vi "15-12-13 UHR-Fleezers Control (host) - 15.2.1UCB Darwin.vi"() -> ()   [LabVIEW 2014] (continued)
            n1711 = Reciprocal(x="Flush rate (uL/m) P3") -> (1/x=w2555:dbl)
            n1712 = Number To Decimal String(number="Volume (uL) P3") -> (decimal integer string=w2560:string)  [unwired: 1 in]
            n1713 = Multiply(x="Volume (uL) P3", y=w2555) -> (x*y=w2554:dbl)
            n1714 = Concatenate Strings("tvolume  " ("string"), w2560, " u" ("string"), "\r") -> (w2558:string)
            n1715 = Multiply(x=w2554, y=60.0) -> (x*y=→"HP3 Flush Time (s)":dbl)
            n1716 = VISA Write(VISA resource name=w2569, write buffer=w2558) -> (VISA resource name out=w2557:refnum<visa-resource-name>)  [unwired: 1 in, 2 out]
            n1717 = Concatenate Strings("cvolume" ("string"), "\r") -> (w2556:string)
            n1718 = VISA Write(VISA resource name=w2557, write buffer=w2556) -> (VISA resource name out=w2567:refnum<visa-resource-name>)  [unwired: 1 in, 2 out]
            n1719 = Concatenate Strings("irun" ("string"), "\r") -> (w2565:string)
            n1720 = VISA Write(VISA resource name=w2567, write buffer=w2565) -> ()  [unwired: 1 in, 3 out]
          }
          frame #1 {
            "Flushing P3" <- TRUE ("Flushing P3")
          }
        }
        n1721 = local read "Save Event Log?"() -> (w2534:bool)
        n1722 = local read "Saving..."() -> (w2535:bool)
        n1723 = And(x=w2534, y=w2535) -> (x .and. y?=w2533:bool)
        n1724 = case shown="True" w2533 {
          tunnel: w2532 -> [_ w2539]
          tunnel: w2531 -> [_ w2538]
          frame False {
          }
          frame True {
            n1725 = Number To Decimal String(number=w2538) -> (decimal integer string=w2543:string)  [unwired: 1 in]
            n1726 = Number To Decimal String(number=w2539) -> (decimal integer string=w2545:string)  [unwired: 1 in]
            n1727 = local read "log file ref"() -> (w2540:refnum<file>)
            n1728 = local read "Time (s)"() -> (w2541:dbl)
            n1729 = Concatenate Strings("pump 3 flushing ", w2543, " uL at ", w2545, " ul/min") -> (w2547:string)
            n1730 = call "write to event log.vi"("log file ref"=w2540, "time"=w2541, "input string"=w2547) -> ()  [unwired: 8 in]
          }
        }
      }
      event "Flush Pump 1": Value Change {
        n1731 = event-data() -> ()  [unwired: 7 out]
        n1732 = flat-sequence {
          tunnel: [w2602] -> w2582
          tunnel: w2581 -> [w2597]
          tunnel: ["Volume (uL) P1"] -> w2577
          tunnel: ["Flush rate (uL/m) P1"] -> w2576
          tunnel: w2582 -> [_]
          frame #0 {
            # "set paramaters (rate, volume) for flush, clear volume"
            n1733 = local write "Inject Pump 1"(TRUE ("Inject Pump 1")) -> ()
            n1734 = Number To Decimal String(number="Flush rate (uL/m) P1") -> (decimal integer string=w2618:string)  [unwired: 1 in]
            n1735 = Concatenate Strings("irate  " ("string"), w2618, " u/m" ("string"), "\r") -> (w2620:string)
            n1736 = VISA Write(VISA resource name=w2597, write buffer=w2620) -> (VISA resource name out=w2616:refnum<visa-resource-name>)  [unwired: 1 in, 2 out]
            n1737 = Reciprocal(x="Flush rate (uL/m) P1") -> (1/x=w2601:dbl)
            n1738 = Number To Decimal String(number="Volume (uL) P1") -> (decimal integer string=w2607:string)  [unwired: 1 in]
            n1739 = Multiply(x="Volume (uL) P1", y=w2601) -> (x*y=w2600:dbl)
            n1740 = Concatenate Strings("tvolume  " ("string"), w2607, " u" ("string"), "\r") -> (w2605:string)
            n1741 = Multiply(x=w2600, y=60.0) -> (x*y=→"HP1 Flush Time (s)":dbl)
            n1742 = VISA Write(VISA resource name=w2616, write buffer=w2605) -> (VISA resource name out=w2604:refnum<visa-resource-name>)  [unwired: 1 in, 2 out]
            n1743 = Concatenate Strings("cvolume" ("string"), "\r") -> (w2603:string)
            n1744 = VISA Write(VISA resource name=w2604, write buffer=w2603) -> (VISA resource name out=w2614:refnum<visa-resource-name>)  [unwired: 1 in, 2 out]
            n1745 = Concatenate Strings("irun" ("string"), "\r") -> (w2612:string)
            n1746 = VISA Write(VISA resource name=w2614, write buffer=w2612) -> (VISA resource name out=w2602:refnum<visa-resource-name>)  [unwired: 1 in, 2 out]
          }
          frame #1 {
            "Flushing P1" <- TRUE ("Flushing P3")
          }
        }
        n1747 = local read "Saving..."() -> (w2578:bool)
        n1748 = local read "Save Event Log?"() -> (w2579:bool)
        n1749 = And(x=w2579, y=w2578) -> (x .and. y?=w2580:bool)
        n1750 = case shown="True" w2580 {
          tunnel: w2577 -> [_ w2586]
          tunnel: w2576 -> [_ w2585]
          frame False {
          }
          frame True {
            n1751 = Number To Decimal String(number=w2586) -> (decimal integer string=w2590:string)  [unwired: 1 in]
            n1752 = Number To Decimal String(number=w2585) -> (decimal integer string=w2588:string)  [unwired: 1 in]
            n1753 = local read "log file ref"() -> (w2592:refnum<file>)
            n1754 = local read "Time (s)"() -> (w2593:dbl)
            n1755 = Concatenate Strings("pump 1 flushing ", w2590, " uL at ", w2588, " ul/min") -> (w2584:string)
            n1756 = call "write to event log.vi"("log file ref"=w2592, "time"=w2593, "input string"=w2584) -> ()  [unwired: 8 in]
          }
        }
      }
      event "Clear Volume": Value Change {
        n1757 = event-data() -> ()  [unwired: 7 out]
        n1758 = Concatenate Strings("cvolume" ("string"), "\r") -> (w2624:string)
        n1759 = VISA Write(VISA resource name=w2623, write buffer=w2624) -> ()  [unwired: 1 in, 3 out]
      }
      event "Clear Volume P3": Value Change {
        n1760 = event-data() -> ()  [unwired: 7 out]
        n1761 = Concatenate Strings("cvolume" ("string"), "\r") -> (w2630:string)
        n1762 = VISA Write(VISA resource name=w2629, write buffer=w2630) -> ()  [unwired: 1 in, 3 out]
        n1763 = local write "Clear Volume P3"(FALSE ("Clear Volume P3")) -> ()
      }
      event "Clear Volume P1": Value Change {
        n1764 = event-data() -> ()  [unwired: 7 out]
        n1765 = Concatenate Strings("cvolume" ("string"), "\r") -> (w2635:string)
        n1766 = local write "Clear Volume P1"(FALSE ("Clear Volume P1")) -> ()
        n1767 = VISA Write(VISA resource name=w2634, write buffer=w2635) -> ()  [unwired: 1 in, 3 out]
      }
      event "Display On P3": Value Change {
        n1768 = event-data() -> ()  [unwired: 7 out]
        n1769 = Select(t="dim 100", s="Display On P3", f="dim 0") -> (s? t:f=w2641:string)
        n1770 = Concatenate Strings(w2641, "\r") -> (w2643:string)
        n1771 = VISA Write(VISA resource name=w2638, write buffer=w2643) -> ()  [unwired: 1 in, 3 out]
      }
      event "Display On P1": Value Change {
        n1772 = event-data() -> ()  [unwired: 7 out]
        n1773 = Select(t="dim 100", s="Display On P1", f="dim 0") -> (s? t:f=w2648:string)
        n1774 = Concatenate Strings(w2648, "\r") -> (w2650:string)
        n1775 = VISA Write(VISA resource name=w2645, write buffer=w2650) -> ()  [unwired: 1 in, 3 out]
      }
      event "Retract Pump 3": Value Change {
        n1776 = event-data() -> ()  [unwired: 7 out]
        n1777 = local write "Retract Pump 3"(FALSE ("Retract Pump 3")) -> ()
        n1778 = case shown="True" "Retract Pump 3" {
          tunnel: w2652 -> [_ w2655]
          frame False {
          }
          frame True {
            n1779 = Number To Decimal String(number="Retract Rate (uL/m)") -> (decimal integer string=w2673:string)  [unwired: 1 in]
            n1780 = Concatenate Strings("wrate  " ("string"), w2673, " u/m" ("string"), "\r") -> (w2675:string)
            n1781 = VISA Write(VISA resource name=w2655, write buffer=w2675) -> (VISA resource name out=w2666:refnum<visa-resource-name>)  [unwired: 1 in, 2 out]
            n1782 = Number To Decimal String(number="Retract Vol 3 (uL)") -> (decimal integer string=w2668:string)  [unwired: 1 in]
            n1783 = Concatenate Strings("tvolume  " ("string"), w2668, " u" ("string"), "\r") -> (w2665:string)
            n1784 = VISA Write(VISA resource name=w2666, write buffer=w2665) -> (VISA resource name out=w2661:refnum<visa-resource-name>)  [unwired: 1 in, 2 out]
            n1785 = Concatenate Strings("cvolume" ("string"), "\r") -> (w2662:string)
            n1786 = VISA Write(VISA resource name=w2661, write buffer=w2662) -> (VISA resource name out=w2656:refnum<visa-resource-name>)  [unwired: 1 in, 2 out]
            n1787 = Concatenate Strings("wrun" ("string"), "\r") -> (w2657:string)
            n1788 = VISA Write(VISA resource name=w2656, write buffer=w2657) -> ()  [unwired: 1 in, 3 out]
          }
        }
      }
      event "Retract Pump 1": Value Change {
        n1789 = event-data() -> ()  [unwired: 7 out]
        n1790 = local write "Retract Pump 1"(FALSE ("Retract Pump 1")) -> ()
        n1791 = case shown="True" "Retract Pump 1" {
          tunnel: w2677 -> [_ w2682]
          frame False {
          }
          frame True {
            n1792 = local read "Retract Rate (uL/m)"() -> (w2680:dbl)
            n1793 = Number To Decimal String(number=w2680) -> (decimal integer string=w2698:string)  [unwired: 1 in]
            n1794 = Concatenate Strings("wrate  " ("string"), w2698, " u/m" ("string"), "\r") -> (w2700:string)
            n1795 = VISA Write(VISA resource name=w2682, write buffer=w2700) -> (VISA resource name out=w2692:refnum<visa-resource-name>)  [unwired: 1 in, 2 out]
            n1796 = Number To Decimal String(number="Retract Vol 1 (uL)") -> (decimal integer string=w2694:string)  [unwired: 1 in]
            n1797 = Concatenate Strings("tvolume  " ("string"), w2694, " u" ("string"), "\r") -> (w2691:string)
            n1798 = VISA Write(VISA resource name=w2692, write buffer=w2691) -> (VISA resource name out=w2688:refnum<visa-resource-name>)  [unwired: 1 in, 2 out]
            n1799 = Concatenate Strings("cvolume" ("string"), "\r") -> (w2689:string)
            n1800 = VISA Write(VISA resource name=w2688, write buffer=w2689) -> (VISA resource name out=w2683:refnum<visa-resource-name>)  [unwired: 1 in, 2 out]
            n1801 = Concatenate Strings("wrun" ("string"), "\r") -> (w2684:string)
            n1802 = VISA Write(VISA resource name=w2683, write buffer=w2684) -> ()  [unwired: 1 in, 3 out]
          }
        }
      }
      event "Flip Green Filter": Value Change {
        n1803 = event-data() -> ()  [unwired: 7 out]
        n1804 = Not(x="Flip Green Filter") -> (.not. x?=w2703:bool)
        n1805 = local write "Flip Green Filter"(w2703) -> ()
        n1806 = flat-sequence {
          tunnel: [w2712] -> w2708
          tunnel: [w2711] -> w2707
          tunnel: w2702 -> [w2710]
          tunnel: [w2715] -> w2706
          tunnel: w2708 -> [w2715]
          tunnel: [w2714] -> w2705
          tunnel: w2707 -> [w2714]
          tunnel: w2706 -> [w2719]
          tunnel: w2705 -> [w2718]
          tunnel: [w2717] -> w2709
          frame #0 {
            n1807 = xnode "Read/Write Control"("FPGA VI Reference In"=w2710, "Green Filter Flipper"=TRUE) -> ("FPGA VI Reference Out"=w2712:T24, "error out"=w2711:errorcluster)  [unwired: 1 in]
          }
          frame #1 {
            n1808 = Wait (ms)(milliseconds to wait=u32 100) -> ()  [unwired: 1 out]
          }
          frame #2 {
            n1809 = xnode "Read/Write Control"("FPGA VI Reference In"=w2719, "error in"=w2718, "Green Filter Flipper"=FALSE) -> ("error out"=w2717:errorcluster)  [unwired: 1 out]
          }
        }
      }
      event "Pump 1 contents", "Pump 3 contents": Value Change {
        n1810 = event-data() -> ()  [unwired: 7 out]
        n1811 = local read "Pump 1 contents"() -> (→"Pump 1 cont disp":string)
        n1812 = local read "Pump 3 contents"() -> (→"Pump 3 cont disp":string)
      }
      event "Reset Trap Pos. FB": Value Change {
        n1813 = event-data() -> ()  [unwired: 7 out]
        n1814 = xnode "Read/Write Control"("FPGA VI Reference In"=w2723, "Trap Pos. FB Reset"="Reset Trap Pos. FB") -> ()  [unwired: 1 in, 2 out]
      }
      event "Rem fb disp offset": Value Change {
        n1815 = event-data() -> ()  [unwired: 7 out]
        n1816 = local write "Rem fb disp offset"(FALSE ("Rem fb disp offset")) -> ()
        n1817 = local read "Mean T1 Position (nm)"() -> (w2726:dbl)
        n1818 = local read "FB Trap Pos Offset"() -> (w2727:dbl)
        n1819 = Subtract(x=w2727, y=w2726) -> (x-y=w2725:dbl)
        n1820 = local write "FB Trap Pos Offset"(w2725) -> ()
      }
      event "Threshold (nm)": Value Change {
        n1821 = event-data() -> ()  [unwired: 7 out]
        n1822 = flat-sequence {
          tunnel: [w2732] -> w2730
          tunnel: w2729 -> [w2731]
          tunnel: w2730 -> [w2743]
          frame #0 {
            n1823 = xnode "Read/Write Control"("FPGA VI Reference In"=w2731) -> ("FPGA VI Reference Out"=w2735:T24, "error out"=w2734:errorcluster, "FPGA TTrig Thresh"=w2736:i64)  [unwired: 1 in]
            n1824 = local read "Threshold stored (nm)"() -> (w2742:dbl)
            n1825 = local read "Threshold (nm)"() -> (w2732:dbl)
            n1826 = local read "AOM X Cal (nm/MHz)"() -> (w2740:dbl)
            n1827 = Subtract(x=w2732, y=w2742) -> (x-y=w2741:dbl)
            n1828 = Divide(x=w2741, y=w2740) -> (x/y=w2738:dbl)
            n1829 = call "IR AOM freq to word.vi"("Frequency In (MHz)"=w2738) -> ("Frequency Word Out (double)"=w2739:dbl)
            n1830 = To Quad Integer(1:w2739) -> (0:w2737:i64)
            n1831 = Add(x=w2736, y=w2737) -> (x+y=w2733:i64)
            n1832 = xnode "Read/Write Control"("FPGA VI Reference In"=w2735, "error in"=w2734, "FPGA TTrig Thresh"=w2733) -> ()  [unwired: 2 out]
          }
          frame #1 {
            "Threshold stored (nm)" <- w2743
          }
        }
      }
      event "FB Trig Integrate": Value Change {
        n1833 = event-data() -> ()  [unwired: 7 out]
        n1834 = local read "FB Trig Integrate"() -> (w2746:u32)
        n1835 = xnode "Read/Write Control"("FPGA VI Reference In"=w2744, "FB Trig Integrate"=w2746) -> ("error out"=w2745:errorcluster)  [unwired: 1 in, 1 out]
      }
      event "11": Value Change {
        n1836 = event-data() -> ()  [unwired: 7 out]
        n1837 = local read "11"() -> (w2747:bool)
        n1838 = case shown="True" w2747 {
          frame False {
          }
          frame True {
            n1839 = local read "Messages"() -> (w2749:string)
            n1840 = call "Update messages.vi"("Message to add"="You kicked it up to 11!", "Old message string"=w2749) -> ("New message string"=w2750:string)
            n1841 = call <vilib>:"Beep.vi"() -> ()  [unwired: 12 in]
            n1842 = local write "Messages"(w2750) -> ()
          }
        }
      }
      event "Trap Pos. FB ON": Value Change {
        n1843 = event-data() -> ()  [unwired: 7 out]
        n1844 = xnode "Read/Write Control"("FPGA VI Reference In"=w2751, "Force feedback"="Trap Pos. FB ON") -> ()  [unwired: 1 in, 2 out]
      }
      event "Remove Action Offset": Value Change {
        n1845 = event-data() -> ()  [unwired: 7 out]
        n1846 = local write "Remove Action Offset"(FALSE ("Remove Action Offset")) -> ()
        n1847 = local read "Trap Pos. FB Mult Factor"() -> (w2758:i64)
        n1848 = local read "Trap Pos FB Action"() -> (w2756:i64)
        n1849 = local read "Trap Pos. FB Offset Factor"() -> (w2754:i64)
        n1850 = Multiply(x=w2758, y=w2756) -> (x*y=w2757:i64)
        n1851 = Add(x=w2757, y=w2754) -> (x+y=w2755:i64)
        n1852 = local write "Trap Pos. FB Offset Factor"(w2755) -> ()
        n1853 = xnode "Read/Write Control"("FPGA VI Reference In"=w2753, "Trap Pos. FB Offset Factor"=w2755) -> ()  [unwired: 1 in, 2 out]
      }
      event "Remove Unwinding Offset": Value Change {
        n1854 = event-data() -> ()  [unwired: 7 out]
        n1855 = local write "Remove Unwinding Offset"(FALSE ("Remove Action Offset")) -> ()
        n1856 = local read "Trap Pos. FB Mult Factor"() -> (w2772:i64)
        n1857 = local read "Trap Pos FB Action"() -> (w2770:i64)
        n1858 = local read "Trap Pos. FB Offset Factor"() -> (w2769:i64)
        n1859 = Multiply(x=w2772, y=w2770) -> (x*y=w2771:i64)
        n1860 = local read "Trap Pos. FB Mult Factor"() -> (w2768:i64)
        n1861 = Add(x=w2771, y=w2769) -> (x+y=w2762:i64)
        n1862 = Multiply(x=32768, y="factor") -> (x*y=w2765:dbl)
        n1863 = Multiply(x=w2765, y=w2768) -> (x*y=w2767:dbl)
        n1864 = Subtract(x=w2762, y=w2767) -> (x-y=w2766:dbl)
        n1865 = To Quad Integer(1:w2766) -> (0:w2761:i64)
        n1866 = xnode "Read/Write Control"("FPGA VI Reference In"=w2760, "Trap Pos. FB Offset Factor"=w2761) -> ()  [unwired: 1 in, 2 out]
        n1867 = local write "Trap Pos. FB Offset Factor"(w2761) -> ()
      }
      event "Trap Pos. FB Range", "Trap Pos. FB Gains", "Trap Pos. FB Mult Factor", "Trap Pos. FB Offset Factor", "Trap Pos FB Negate Action", "Trap Pos FB Monitor\nT1 or T2", "Differential FB?", "Negate Diff?": Value Change {
        n1868 = event-data() -> ()  [unwired: 7 out]
        n1869 = Unbundle By Name("Trap Pos. FB Gains") -> ("proportional gain (Kc)"=w2777:fxp<+/-,16,8>, "integral gain (Kc*Ts/Ti)"=w2776:fxp<+/-,16,8>, "derivative gain (Kc*Td/Ts)"=w2775:fxp<+/-,16,8>)
        n1870 = local read "Negate Diff?"() -> (w2782:bool)
        n1871 = Unbundle By Name("Trap Pos. FB Range") -> ("output high"=w2780:fxp<+/-,16,1>, "output low"=w2779:fxp<+/-,16,1>)
        n1872 = xnode "Read/Write Control"("FPGA VI Reference In"=w2774, "FB2 output high"=w2780, "FB2 output low"=w2779, "P2"=w2777, "I2"=w2776, "D2"=w2775, "Trap Pos. FB Mult Factor"="Trap Pos. FB Mult Factor", "Trap Pos. FB Offset Factor"="Trap Pos. FB Offset Factor", "Trap Pos FB Negate Action"="Trap Pos FB Negate Action", "Trap Pos FB Monitor T1 or T2"="Trap Pos FB Monitor\nT1 or T2", "AI1 X Scale"="Trap Pos. AI1 X Pre-scale", "Negate Diff?"=w2782, "Diff FB Measurement?"="Differential FB?") -> ()  [unwired: 1 in, 2 out]
      }
      event "Trap Pos FB SP", "Trap Pos FB SP 2", "Use SP 2": Value Change {
        n1873 = event-data() -> ()  [unwired: 7 out]
        n1874 = Select(t="Trap Pos FB SP 2", s="Use SP 2", f="Trap Pos FB SP") -> (s? t:f=w2790:fxp<+/-,16,1>)
        n1875 = xnode "Read/Write Control"("FPGA VI Reference In"=w2789, "Trap Pos. FB SP"=w2790) -> ()  [unwired: 1 in, 2 out]
      }
      event "Offset SP2 from SP1": Value Change {
        n1876 = event-data() -> ()  [unwired: 7 out]
        n1877 = local read "Trap Pos FB SP"() -> (w2796:fxp<+/-,16,1>)
        n1878 = Add(x=w2796, y="SP2 Offset") -> (x+y=w2794:fxp<+/-,16,1>)
        n1879 = property on="Trap Pos FB SP 2" class="DigNum (strict)"("Val(Sgnl)"=w2794) -> ()  [unwired: 2 in, 2 out]
        n1880 = local write "Offset SP2 from SP1"(FALSE ("Offset SP2 from SP1")) -> ()
      }
      event "Set Reading to\nSetpoint": Value Change {
        # "This is the actual PID input signal"
        n1881 = event-data() -> ()  [unwired: 7 out]
        n1882 = local write "Set Reading to\nSetpoint"(FALSE ("Set SP to Reading")) -> ()
        n1883 = xnode "Read/Write Control"("FPGA VI Reference In"=w2798) -> ("FPGA VI Reference Out"=w2801:T24, "error out"=w2800:errorcluster, "Trap Pos FB Int-Norm Signal"=w2799:fxp<+/-,16,1>)  [unwired: 1 in]
        n1884 = local read "Differential FB?"() -> (w2802:bool)
        n1885 = case shown="False" w2802 {
          tunnel: [w2807 w2814] -> w2804
          tunnel: w2799 -> [w2805 w2814]
          frame False {
            n1886 = local read "Trap Pos FB Monitor\nT1 or T2"() -> (w2810:bool)
            n1887 = local read "Trap X AI1 (DMA)"() -> (w2813:T15)
            n1888 = Unbundle By Name(w2813) -> ("Set 1"=w2812:fxp<+/-,16,1>, "Set 2"=w2811:fxp<+/-,16,1>)
            n1889 = Select(t=w2812, s=w2810, f=w2811) -> (s? t:f=w2809:fxp<+/-,16,1>)
            n1890 = Not(x="Set SP Using...") -> (.not. x?=w2806:bool)
            n1891 = Select(t=w2805, s=w2806, f=w2809) -> (s? t:f=w2807:fxp<+/-,16,1>)
          }
          frame True {
          }
        }
        n1892 = xnode "Read/Write Control"("FPGA VI Reference In"=w2801, "error in"=w2800, "Trap Pos. FB SP"=w2804) -> ()  [unwired: 2 out]
        n1893 = local write "Trap Pos FB SP"(w2804) -> ()
      }
      event "Trap Pos. FB Out Scale 2^n": Value Change {
        n1894 = event-data() -> ()  [unwired: 7 out]
        n1895 = Scale By Power Of 2(n="Trap Pos. FB Out Scale 2^n", x=ext 1.0) -> (x*2^n=w2815:ext)
        n1896 = property on="Trap Pos. FB Mult Factor" class="DigNum (strict)"("Val(Sgnl)"=w2815) -> ()  [unwired: 2 in, 2 out]
      }
      event "Trap Pos FB Int Count": Value Change {
        n1897 = event-data() -> ()  [unwired: 7 out]
        n1898 = xnode "Read/Write Control"("FPGA VI Reference In"=w2818, "Trap Pos FB Int Count"="Trap Pos FB Int Count") -> ()  [unwired: 1 in, 2 out]
      }
      event "Display Saved Data": Value Change {
        n1899 = event-data() -> ()  [unwired: 7 out]
        n1900 = case shown="\"Amp Current\"" "Display Saved Data" {
          frame "Bead Seperation", Default {
            n1901 = property on="Amp current" class="WFGraph (strict)"("Visible"=FALSE) -> ()  [unwired: 2 in, 2 out]
            n1902 = property on="Trap Delta Graph" class="WFGraph (strict)"("Visible"=TRUE) -> ()  [unwired: 2 in, 2 out]
            n1903 = property on="Saved trap pos" class="WFGraph (strict)"("Visible"=FALSE) -> ()  [unwired: 2 in, 2 out]
          }
          frame "Amp Current" {
            n1904 = property on="Saved trap pos" class="WFGraph (strict)"("Visible"=FALSE) -> ()  [unwired: 2 in, 2 out]
            n1905 = property on="Trap Delta Graph" class="WFGraph (strict)"("Visible"=FALSE) -> ()  [unwired: 2 in, 2 out]
            n1906 = property on="Amp current" class="WFGraph (strict)"("Visible"=TRUE) -> ()  [unwired: 2 in, 2 out]
          }
          frame "Trap Position" {
            n1907 = property on="Saved trap pos" class="WFGraph (strict)"("Visible"=TRUE) -> ()  [unwired: 2 in, 2 out]
            n1908 = property on="Trap Delta Graph" class="WFGraph (strict)"("Visible"=FALSE) -> ()  [unwired: 2 in, 2 out]
            n1909 = property on="Amp current" class="WFGraph (strict)"("Visible"=FALSE) -> ()  [unwired: 2 in, 2 out]
          }
        }
      }
      event "Calibration": Value Change {
        n1910 = event-data() -> ()  [unwired: 7 out]
        n1911 = local read "X or Y?"() -> (w2846:bool)
        n1912 = local read "Calibration"() -> (w2843:u16)
        n1913 = Select(t="X" ("Label.Text"), s=w2846, f="Y" ("Label.Text")) -> (s? t:f=w2840:string)
        n1914 = case shown="0, Default" w2843 {
          tunnel: ["Position (V)" ("Label.Text") "Position (nm)" ("Label.Text") "Force (pN)" ("Label.Text")] -> w2837
          tunnel: [" (V)" ("Label.Text") " (nm)" ("Label.Text") " (pN)" ("Label.Text")] -> w2834
          frame 0, Default {
          }
          frame 1 {
          }
          frame 2 {
          }
        }
        n1915 = Concatenate Strings("T1 " ("Label.Text"), w2840) -> (w2836:string)
        n1916 = Concatenate Strings("T2 " ("Label.Text"), w2840) -> (w2835:string)
        n1917 = property on="Force" class="WFChart (strict)"("YScale.NameLbl.Text"=w2837) -> ()  [unwired: 2 in, 2 out]
        n1918 = Concatenate Strings("Mean" ("Label.Text"), w2834) -> (w2833:string)
        n1919 = Concatenate Strings(w2836, w2834) -> (w2832:string)
        n1920 = Concatenate Strings(w2835, w2834) -> (w2831:string)
        n1921 = Concatenate Strings("Difference" ("Label.Text"), w2834) -> (w2830:string)
        n1922 = property on="Mean" class="DigNum (strict)"("Caption.Text"=w2833) -> ()  [unwired: 2 in, 2 out]
        n1923 = property on="T1 X" class="DigNum (strict)"("Caption.Text"=w2832) -> ()  [unwired: 2 in, 2 out]
        n1924 = property on="T2 X" class="DigNum (strict)"("Caption.Text"=w2831) -> ()  [unwired: 2 in, 2 out]
        n1925 = property on="Difference" class="DigNum (strict)"("Caption.Text"=w2830) -> ()  [unwired: 2 in, 2 out]
      }
      event "Base N trap periods", "Period scale factor", "Trap osc amp (MHz)", "Cal sets to save", "# Samples/trap", "Total Counts (ticks)": Value Change {
        w2853 = 1.0
        w2859 = u32 0 ("y")
        # "scales 0 to 2pi"
        # "Create vector of trap offset (oscillation) values."
        # "Compute oscillation period as a multiple of the trap period. Should also fit nicely as a factor of the DMA period.\nCompare ticks for accurate commensurability check."
        # "Oscillation frequency needs to be commensurate\nwith the data save time."
        # "Be commensurate with total save time/100 (or so). That way you are guaranteed you can average spectra at least 100x."
        n1926 = event-data() -> ()  [unwired: 7 out]
        n1927 = local read "Total Counts (ticks)"() -> (w2875:u16)
        n1928 = To Unsigned Long Integer(number=w2875) -> (unsigned 32bit integer=w2885:u32)
        n1929 = Multiply "Base osc period (ticks)"(x=w2885, y="Base N trap periods") -> (x*y=w2876:u32)
        n1930 = local read "# Samples/trap"() -> (w2880:u32)
        n1931 = Multiply "Scaled osc period (ticks)"(x=w2876, y="Period scale factor") -> (x*y=w2877:dbl)
        n1932 = Multiply(x="Base N trap periods", y="Period scale factor") -> ()  [unwired: 1 out]
        n1933 = local read "Cal sets to save"() -> (w2881:u32)
        n1934 = To Unsigned Quad Integer(1:w2877) -> (0:w2867:u64)
        n1935 = for "vector 0 to N -1" {
          N: w2853 -> [_]
          tunnel: [w2902] -> w2873 mode=indexing
          i -> [w2902]
        }
        n1936 = Multiply "Ticks/DMA"(x=w2880, y=w2885) -> (x*y=w2884:u32)
        n1937 = Multiply "Scaled osc period (s)"(x=w2867, y=2.5e-08) -> (x*y=w2879:dbl)
        "Trap OSC Period (s)" <- w2879
        n1938 = Reciprocal(x=w2879) -> (1/x=→"A cal freq (Hz)":dbl)
        n1939 = Multiply(x=w2873, y=6.283185307179586) -> (x*y=w2888:dbl[])
        n1940 = Quotient & Remainder(x=w2884, y=w2867) -> (x-y*floor(x/y)=w2860:u64, floor(x/y)=→"N osc / DMA":u64)
        "DMA remainder" <- w2860
        n1941 = Multiply "Total trap ticks"(x=w2881, y=w2884) -> (x*y=w2868:u32)
        n1942 = Divide(x=w2888, y=w2853) -> (x/y=w2889:dbl[])
        n1943 = Sine(x=w2889) -> (sin(x)=w2890:dbl[])
        n1944 = Quotient & Remainder(x=w2868, y=100) -> (x-y*floor(x/y)=w2863:u32, floor(x/y)=w2883:u32)
        "Total save/100 remainder" <- w2863
        n1945 = Multiply "Single period osc vector"(x=w2890, y="Trap osc amp (MHz)") -> (x*y=w2866:dbl[])
        n1946 = Quotient & Remainder(x=w2883, y=w2867) -> (x-y*floor(x/y)=w2862:u64, floor(x/y)=→"N osc/ (total save/100)":u64)
        "(total save/100) /osc period remainder" <- w2862
        n1947 = Quotient & Remainder(x=w2868, y=w2867) -> (x-y*floor(x/y)=w2861:u64)  [unwired: 1 out]
        "N trap osc periods per save remainder" <- w2861
        n1948 = call "IR AOM freq to word - vec.vi"("Frequency In (double vec, MHz)"=w2866) -> ("Frequency Word Out"=w2865:dbl[])
        n1949 = To Quad Integer(1:w2865) -> (0:w2864:i64[])
        n1950 = disable-structure shown="Disabled" {
          disable-tunnel: w2872 -> [w2894 _]
          disable-tunnel: w2864 -> [w2892 _]
          frame Disabled {
            n1951 = xnode "Read/Write Control"("FPGA VI Reference In"=w2894) -> ("FPGA VI Reference Out"=w2893:T24)  [unwired: 3 in, 1 out]
            n1952 = flat-sequence {
              tunnel: w2892 -> [w2897]
              tunnel: w2893 -> [w2896]
              frame #0 {
                n1953 = for "Write data to fpga memory" {
                  tunnel: w2896 -> [w2899]
                  tunnel: w2897 -> [_] mode=indexing
                  (unwired) TRUE ("Ready Write")
                  n1954 = xnode "Read/Write Control"("FPGA VI Reference In"=w2899) -> ("FPGA VI Reference Out"=w2898:T24)  [unwired: 4 in, 1 out]
                  n1955 = while {
                    tunnel: w2898 -> [w2900]
                    stop <- _ continue-if-true
                    n1956 = xnode "Read/Write Control"("FPGA VI Reference In"=w2900) -> ()  [unwired: 1 in, 3 out]
                  }
                }
                "Writing waveform to fpga memory" <- TRUE ("Writing waveform to fpga memory")
              }
              frame #1 {
                n1957 = local write "Writing waveform to fpga memory"(FALSE ("Writing waveform to fpga memory")) -> ()
              }
            }
          }
          frame Enabled {
          }
        }
        n1958 = Equal?(x=w2862, y=w2859) -> (x = y?=w2857:bool)
        n1959 = Equal?(x=w2863, y=w2859) -> (x = y?=w2858:bool)
        n1960 = Equal?(x=w2860, y=w2859) -> (x = y?=w2855:bool)
        n1961 = Equal?(x=w2861, y=w2859) -> (x = y?=w2856:bool)
        n1962 = Compound Arithmetic op=AND(w2858, w2857, w2856, w2855) -> (→"Good freq?":bool)
      }
      event "Osc trap cont.", "Osc traps", "T1 Osc Enable", "T2 Osc Enable": Value Change {
        n1963 = event-data() -> ()  [unwired: 7 out]
        n1964 = xnode "Read/Write Control"("FPGA VI Reference In"=w2905, "Trap 1 osc enable"="T1 Osc Enable", "Trap 2 osc enable"="T2 Osc Enable") -> ()  [unwired: 1 in, 2 out]
      }
      event "Pressure Pump Voltage (+/-10V)": Value Change {
        n1965 = event-data() -> ()  [unwired: 7 out]
        n1966 = disable-structure shown="Disabled" {
          disable-tunnel: w2906 -> [w2910 _]
          frame Disabled {
            n1967 = Divide(x="Pressure Pump Voltage (+/-10V)", y=10.0) -> (x/y=w2907:dbl)
            n1968 = Multiply(x=w2907, y=32767.0) -> (x*y=w2908:dbl)
            n1969 = xnode "Read/Write Control"("FPGA VI Reference In"=w2910, "Pressure Pump"=w2908) -> ()  [unwired: 1 in, 2 out]
          }
          frame Enabled {
          }
        }
      }
    }
    "error out 2" <- w1526
    n1970 = node-c288() -> ()  [unwired: 2 out]
  }
  n1971 = node-c288() -> (w61:T27)  [unwired: 4 out]
  n1972 = timed-loop "Mouse control: trap position (AOM deflection), set confocal spot from image" {
    tunnel: [w2914] -> w66
    timing: w61 -> [_]
    timing-out: [_] -> w60
    tunnel: w15 -> [w2913]
    stop <- w2914 stop-if-true
    n1973 = node-c288() -> ()  [unwired: 2 out]
    n1974 = event shown="[0] \"Pane\": Mouse Down" {
      selector: _ -> [_ _]
      dyn-events: _ -> [_ _]
      timeout: _ -> [_ _]
      tunnel: w2913 -> [w2917 _]
      event Mouse Down {
        n1975 = event-data() -> ("Time"=w2919:u32, "Coords"=w2918:T9, "Button"=w2920:u16)  [unwired: 6 out]
        n1976 = case shown="3" w2920 {
          tunnel: w2919 -> [_ _ w3026]
          tunnel: w2918 -> [_ w2957 w3024]
          tunnel: w2917 -> [_ _ w3020]
          frame 0, Default {
          }
          frame 1 {
            n1977 = property on="APD 2" class="ImageControl"() -> ("Displayed Image Position"=w2927:cluster{"Left":i32, "Top":i32})  [unwired: 2 in, 2 out]
            n1978 = property on="APD 1" class="ImageControl"() -> ("Displayed Image Position"=w2956:cluster{"Left":i32, "Top":i32})  [unwired: 2 in, 2 out]
            n1979 = property on="Detection Laser X" class="ImageControl"() -> ("Displayed Image Position"=w2953:cluster{"Left":i32, "Top":i32})  [unwired: 2 in, 2 out]
            n1980 = property on="Detection Laser Y" class="ImageControl"() -> ("Displayed Image Position"=w2952:cluster{"Left":i32, "Top":i32})  [unwired: 2 in, 2 out]
            n1981 = property on="APD 2" class="ImageControl"() -> ("Displayed Image Size"=w2926:cluster{"Width":u32, "Height":u32})  [unwired: 2 in, 2 out]
            n1982 = property on="APD 1" class="ImageControl"() -> ("Displayed Image Size"=w2954:cluster{"Width":u32, "Height":u32})  [unwired: 2 in, 2 out]
            n1983 = property on="Detection Laser X" class="ImageControl"() -> ("Displayed Image Size"=w2955:cluster{"Width":u32, "Height":u32})  [unwired: 2 in, 2 out]
            n1984 = property on="Detection Laser Y" class="ImageControl"() -> ("Displayed Image Size"=w2951:cluster{"Width":u32, "Height":u32})  [unwired: 2 in, 2 out]
            n1985 = Unbundle By Name(w2926) -> ("Width"=w2923:u32, "Height"=w2922:u32)
            n1986 = Unbundle By Name(w2927) -> ("Left"=w2925:i32, "Top"=w2924:i32)
            n1987 = Unbundle By Name(w2954) -> ("Width"=w2948:u32, "Height"=w2947:u32)
            n1988 = Unbundle By Name(w2955) -> ("Width"=w2944:u32, "Height"=w2943:u32)
            n1989 = Unbundle By Name(w2951) -> ("Width"=w2940:u32, "Height"=w2939:u32)
            n1990 = Unbundle By Name(w2956) -> ("Left"=w2950:i32, "Top"=w2949:i32)
            n1991 = Unbundle By Name(w2953) -> ("Left"=w2946:i32, "Top"=w2945:i32)
            n1992 = Unbundle By Name(w2952) -> ("Left"=w2942:i32, "Top"=w2941:i32)
            n1993 = Bundle("Left"=w2925, "Top"=w2924, "Width"=w2923, "Height"=w2922) -> (w2921:T37)  [unwired: 1 in]
            n1994 = Bundle("Left"=w2950, "Top"=w2949, "Width"=w2948, "Height"=w2947) -> (w2938:T37)  [unwired: 1 in]
            n1995 = Bundle("Left"=w2946, "Top"=w2945, "Width"=w2944, "Height"=w2943) -> (w2937:T37)  [unwired: 1 in]
            n1996 = Bundle("Left"=w2942, "Top"=w2941, "Width"=w2940, "Height"=w2939) -> (w2936:T37)  [unwired: 1 in]
            n1997 = Build Cluster Array(w2921, w2938, w2937, w2936) -> (w2935:T38)
            n1998 = for {
              tunnel: w2957 -> [w2968]
              tunnel: w2935 -> [w2969] mode=indexing
              shift-right: [w2966] -> w2933
              shift-left: TRUE -> [w2967]
              shift-right: [w2965] -> w2931
              shift-left: _ -> [w2961]
              shift-right: [w2964] -> w2930
              shift-left: _ -> [w2960]
              shift-right: [w2963] -> w2929
              shift-left: _ -> [w2959]
              shift-right: [w2962] -> w2928
              shift-left: _ -> [w2958]
              n1999 = case shown="True" w2967 {
                selector: w2967 -> [w2974 _]
                tunnel: w2969 -> [_ w2983]
                tunnel: w2968 -> [_ w2981]
                tunnel: [w2974 w2979] -> w2966
                tunnel: [w2973 w2978] -> w2965
                tunnel: [w2972 w2977] -> w2964
                tunnel: [w2971 w2976] -> w2963
                tunnel: [w2970 w2975] -> w2962
                tunnel: w2961 -> [w2973 _]
                tunnel: w2960 -> [w2972 _]
                tunnel: w2959 -> [w2971 _]
                tunnel: w2958 -> [w2970 _]
                frame False {
                }
                frame True {
                  n2000 = Unbundle(w2983) -> (w2982:T37)
                  n2001 = call "isclickinwindow.vi"("Image Param"=w2982, "Point32"=w2981) -> ("4 Y"=w2975:i32, "3 Height"=w2976:i32, "2 X"=w2977:i32, "1 Width"=w2978:i32, "In image?"=w2980:bool)  [unwired: 1 in]
                  n2002 = Not(x=w2980) -> (.not. x?=w2979:bool)
                }
              }
            }
            n2003 = Not(x=w2933) -> (.not. x?=w2932:bool)
            n2004 = case shown="True" w2932 {
              tunnel: w2930 -> [_ w2997]
              tunnel: w2928 -> [_ w2996]
              tunnel: w2931 -> [_ w2995]
              tunnel: w2929 -> [_ w2994]
              frame False {
              }
              frame True {
                w2984 = FALSE ("Get Point")
                n2005 = local read "Scan lines (y)"() -> (w2999:u64)
                n2006 = disable-structure shown="Disabled" {
                  frame Disabled {
                  }
                  frame Enabled {
                  }
                }
                n2007 = local read "Actual MCL Inc (V)"() -> (w2993:dbl)
                n2008 = local read "Scan steps (MCL)"() -> (w2998:u64)
                n2009 = Divide "Y Pix/step"(x=w2994, y=w2999) -> (x/y=w3006:dbl)
                n2010 = Divide "Y V/pix"(x=w2993, y=w3006) -> (x/y=w3005:dbl)
                n2011 = Divide "Y half step offset"(x=w2993, y=2.0) -> (x/y=w3007:dbl)
                n2012 = Divide "X pix/step"(x=w2995, y=w2998) -> (x/y=w3004:dbl)
                n2013 = Negate(x=w3007) -> (-x=w3008:dbl)
                n2014 = local read "Initial Y"() -> (w3014:dbl)
                n2015 = Multiply(x=w2996, y=w3005) -> (x*y=w3015:dbl)
                n2016 = Divide "X half step offset"(x=w2993, y=2.0) -> (x/y=w3001:dbl)
                n2017 = Divide "X V/pix"(x=w2993, y=w3004) -> (x/y=w3003:dbl)
                n2018 = Multiply(x=w2993, y=w2998) -> (x*y=w3010:dbl)
                n2019 = Compound Arithmetic op=ADD(w3008, w3015, w3014) -> (w2985:dbl)
                "Pointer Y (V)" <- w2985
                n2020 = Multiply(x=w3003, y=w2997) -> (x*y=w3012:dbl)
                n2021 = Negate(x=w3001) -> (-x=w3000:dbl)
                n2022 = local read "Initial X"() -> (w3013:dbl)
                n2023 = Negate(x=w3012) -> (-x=w3011:dbl)
                n2024 = Compound Arithmetic op=ADD(w3000, w3010, w3013, w3011) -> (w2986:dbl)
                "Pointer X (V)" <- w2986
                n2025 = case shown="True" "Set High F Confocal Spot (X-Y)" {
                  tunnel: w2986 -> [_ w3016]
                  tunnel: w2985 -> [_ w3017]
                  frame False {
                  }
                  frame True {
                    "Confocal Y 2 (V)" <- w3017
                    "Confocal X 2 (V)" <- w3016
                  }
                }
                n2026 = Or(x="Set X Only", y="Set Confocal Spot (X-Y)") -> (x .or. y?=w2989:bool)
                n2027 = Or(x="Set Confocal Spot (X-Y)", y="Set Y Only") -> (x .or. y?=w2988:bool)
                n2028 = case shown="True" w2989 {
                  tunnel: w2986 -> [_ w3018]
                  frame False {
                  }
                  frame True {
                    n2029 = property on="AO2" class="Slide (strict)"("Val(Sgnl)"=w3018) -> ()  [unwired: 2 in, 2 out]
                    "Confocal X 1 (V)" <- w3018
                  }
                }
                n2030 = case shown="True" w2988 {
                  tunnel: w2985 -> [_ w3019]
                  frame False {
                  }
                  frame True {
                    n2031 = property on="AO1" class="Slide (strict)"("Val(Sgnl)"=w3019) -> ()  [unwired: 2 in, 2 out]
                    "Confocal Y 1 (V)" <- w3019
                  }
                }
                n2032 = local write "Set High F Confocal Spot (X-Y)"(w2984) -> ()
                n2033 = local write "Set Confocal Spot (X-Y)"(w2984) -> ()
                n2034 = local write "Set X Only"(w2984) -> ()
                n2035 = local write "Set Y Only"(w2984) -> ()
              }
            }
          }
          frame 3 {
            n2036 = local read "BD 2 Frequency 1 (MHz)"() -> (w3021:dbl)
            n2037 = local read "BD 1 Frequency 1 (MHz)"() -> (w3022:dbl)
            n2038 = local write "Manipulating Trap"(TRUE ("Manipulating Trap")) -> ()
            n2039 = local write "Coords"(T9 {"Horizontal"=0, "Vertical"=0} ("Coords")) -> ()
            n2040 = while {
              tunnel: w3026 -> [w3031]
              tunnel: w3024 -> [w3030]
              tunnel: w3022 -> [w3029]
              tunnel: w3021 -> [w3028]
              tunnel: w3020 -> [w3027]
              stop <- w3032 stop-if-true
              n2041 = event shown="[0] \"Pane\": Mouse Move" {
                selector: _ -> [_ _]
                dyn-events: _ -> [_ _]
                timeout: _ -> [_ _]
                tunnel: ["Force Manip Abort" w3096] -> w3032
                tunnel: w3031 -> [w3039 _]
                tunnel: w3030 -> [w3037 _]
                tunnel: w3029 -> [w3036 _]
                tunnel: w3028 -> [w3035 _]
                tunnel: w3027 -> [w3033 _]
                event Mouse Move {
                  n2042 = event-data() -> ("Time"=w3040:u32, "Coords"=w3041:T9)  [unwired: 3 out]
                  n2043 = Less?(x=w3040, y=w3039) -> (x < y?=w3038:bool)
                  n2044 = case "Makes sure old motion events prior to mouse click aren't used" shown="False" w3038 {
                    tunnel: w3041 -> [w3083 _]
                    tunnel: w3037 -> [w3084 _]
                    tunnel: w3036 -> [w3058 _]
                    tunnel: w3035 -> [w3057 _]
                    tunnel: w3033 -> [w3042 _]
                    frame False {
                      n2045 = Subtract(x=w3083, y=w3084) -> (x-y=w3082:T9)
                      "Coords" <- w3082
                      n2046 = local read "Y RF Frequency Limits (MHz)"() -> (w3043:T18)
                      n2047 = To Double Precision Float(number=w3082) -> (double precision float=w3081:cluster{"Horizontal":dbl, "Vertical":dbl})
                      n2048 = Multiply(x=cluster{"Horizontal":dbl, "Vertical":dbl} {"Horizontal"=-1.0, "Vertical"=1.0}, y="Manipulation Scaling") -> (x*y=w3077:cluster{"Horizontal":dbl, "Vertical":dbl})
                      n2049 = local read "X RF Frequency Limits (MHz)"() -> (w3044:T18)
                      n2050 = Multiply(x=w3081, y=w3077) -> (x*y=w3079:cluster{"Horizontal":dbl, "Vertical":dbl})
                      n2051 = Unbundle By Name(w3079) -> ("Horizontal"=w3074:dbl, "Vertical"=w3078:dbl)
                      n2052 = Unbundle By Name(w3043) -> ("Maximum"=w3046:dbl, "Minimum"=w3045:dbl)
                      n2053 = Boolean To (0,1)(Boolean="Manip. X?") -> (0, 1=w3072:i16)
                      n2054 = Boolean To (0,1)(Boolean="Manip. Y?") -> (0, 1=w3069:i16)
                      n2055 = local read "BD 1 Frequency 2 (MHz)"() -> (w3060:dbl)
                      n2056 = Multiply(x=w3078, y=w3069) -> (x*y=w3071:dbl)
                      n2057 = Multiply(x=w3072, y=w3074) -> (x*y=w3075:dbl)
                      n2058 = local read "BD 2 Frequency 2 (MHz)"() -> (w3059:dbl)
                      n2059 = Unbundle By Name(w3044) -> ("Maximum"=w3048:dbl, "Minimum"=w3047:dbl)
                      n2060 = Add(x=w3057, y=w3071) -> (x+y=w3050:dbl)
                      n2061 = Add(x=w3058, y=w3075) -> (x+y=w3052:dbl)
                      n2062 = In Range and Coerce(upper limit=w3048, x=w3052, lower limit=w3047) -> (coerced(x)=w3051:dbl)  [unwired: 1 out]
                      n2063 = In Range and Coerce(upper limit=w3046, x=w3050, lower limit=w3045) -> (coerced(x)=w3049:dbl)  [unwired: 1 out]
                      n2064 = Subtract(x=w3051, y=w3060) -> (x-y=w3068:dbl)
                      n2065 = Subtract(x=w3049, y=w3059) -> (x-y=w3067:dbl)
                      n2066 = Square(x=w3068) -> (x^2=w3066:dbl)
                      n2067 = Square(x=w3067) -> (x^2=w3065:dbl)
                      n2068 = Add(x=w3066, y=w3065) -> (x+y=w3064:dbl)
                      n2069 = Square Root(x=w3064) -> (sqrt(x)=w3061:dbl)
                      n2070 = In Range and Coerce(upper limit="Limit Max (MHz)", x=w3061, lower limit="Limit Min (MHz)") -> (In Range?=w3054:bool)  [unwired: 1 out]
                      n2071 = Not(x="Limits Enable") -> (.not. x?=w3053:bool)
                      n2072 = Or(x=w3054, y=w3053) -> (x .or. y?=w3055:bool)
                      n2073 = case shown="True" w3055 {
                        tunnel: w3061 -> [_ w3086]
                        tunnel: w3051 -> [_ w3093]
                        tunnel: w3060 -> [_ w3092]
                        tunnel: w3049 -> [_ w3091]
                        tunnel: w3059 -> [_ w3090]
                        tunnel: w3044 -> [_ w3088]
                        tunnel: w3043 -> [_ w3087]
                        tunnel: w3042 -> [_ w3085]
                        frame False {
                        }
                        frame True {
                          n2074 = local read "BD 1 Frequency 3 (MHz)"() -> (w3094:dbl)
                          n2075 = local read "BD 2 Frequency 3 (MHz)"() -> (w3089:dbl)
                          n2076 = local write "Trap Delta (MHz)"(w3086) -> ()
                          n2077 = call "set RF board frequency - interlace.vi"("Board 2 Frequency Limits"=w3087, "Board 1 Frequency Limits"=w3088, "FPGA VI Reference In"=w3085, "Board 2 Frequency 3 (MHz)"=w3089, "Board 1 Frequency 3 (MHz)"=w3094, "Board 2 Frequency 2 (MHz)"=w3090, "Board 2 Frequency 1 (MHz)"=w3091, "Board 1 Frequency 2 (MHz)"=w3092, "Board 1 Frequency 1  (MHz)"=w3093) -> ()  [unwired: 1 in, 2 out]
                          n2078 = local write "BD 2 Frequency 1 (MHz)"(w3091) -> ()
                          n2079 = local write "BD 1 Frequency 1 (MHz)"(w3093) -> ()
                        }
                      }
                    }
                    frame True {
                    }
                  }
                }
                event Mouse Up {
                  n2080 = event-data() -> ("Button"=w3095:u16)  [unwired: 8 out]
                  n2081 = case shown="3" w3095 {
                    tunnel: [FALSE TRUE] -> w3096
                    frame 0, Default {
                    }
                    frame 3 {
                      n2082 = local read "Trap Delta (MHz)"() -> (w3098:dbl)
                      n2083 = property on="Initial delta (MHz)" class="DigNum (strict)"("Val(Sgnl)"=w3098) -> ()  [unwired: 2 in, 2 out]
                      n2084 = local write "Manipulating Trap"(FALSE ("Manipulating Trap")) -> ()
                    }
                  }
                }
              }
            }
          }
        }
      }
      event Mouse Move {
        n2085 = event-data() -> ()  [unwired: 6 out]
      }
    }
    n2086 = local read "Stop All"() -> (w2914:bool)
    n2087 = node-c288() -> ()  [unwired: 2 out]
  }
  n2088 = disable-structure shown="Disabled" {
    frame Disabled {
      n2089 = flat-sequence "Video" {
        tunnel: [w3112] -> w3101
        tunnel: w3101 -> [w3153]
        frame #0 {
          w3102 = FALSE ("File open?")
          n2090 = while {
            stop <- w3104 continue-if-true
            n2091 = call "Close Video Capture.vi"() -> ("error code OUT"=w3106:i32)
            n2092 = Equal?(x=w3106, y=0) -> (x = y?=w3104:bool)
          }
          n2093 = local write "New Video File"(w3102) -> ()
          n2094 = local write "File open?"(w3102) -> ()
          n2095 = local write "Save Video"(w3102) -> ()
          n2096 = local write "Stop All"(FALSE ("Stop All")) -> ()
        }
        frame #1 {
          n2097 = call "DMR_Init.vi"() -> ()  [unwired: 3 out]
        }
        frame #2 {
          w3107 = "DE245428202"  # MSU fleezers card #
          (unwired) "DE019116701"  # Illinois fleezers card #
          # "Setting the destination format to Mono8 makes sure that the image can be displayed in the intensity plot."
          n2098 = call "DMR_GetDevice.vi"("search string IN"=w3107) -> ("device handle OUT"=w3130:i32)  [unwired: 4 in, 2 out]
          n2099 = call "DMR_OpenDevice.vi"("device handle IN"=w3130) -> ("driver handle OUT"=w3113:i32)  [unwired: 4 out]
          n2100 = call "DMR_FindList.vi"("flags IN"=u32 0 ("flags"), "list name IN"="" ("String"), "list type IN"=T39."camera descriptions", "driver handle IN"=w3113) -> ("list handle OUT"=w3116:i32)  [unwired: 2 out]
          n2101 = call "DMR_FindList.vi"("flags IN"=u32 0 ("flags"), "list name IN"="Base", "list type IN"=T39."setting", "driver handle IN"=w3113) -> ("list handle OUT"=w3114:i32)  [unwired: 2 out]
          n2102 = call "OBJ_GetHandle.vi"("object name IN"="VideoStandard", "list handle IN"=w3116) -> ("object handle OUT"=w3110:i32)  [unwired: 3 out]
          n2103 = call "OBJ_GetHandle.vi"("object name IN"="PixelFormat", "list handle IN"=w3114) -> ("object handle OUT"=w3124:i32)  [unwired: 3 out]
          n2104 = call "OBJ_SetS.vi"("value index IN"=0, "value IN"="NTSC M", "object handle IN"=w3110) -> ()  [unwired: 2 out]
          n2105 = call "OBJ_SetS.vi"("value index IN"=0, "value IN"="Mono8" ("value"), "object handle IN"=w3124) -> ()  [unwired: 2 out]
          n2106 = call "OBJ_GetHandle.vi"("object name IN"="VideoChannel", "list handle IN"=w3114) -> ("object handle OUT"=w3120:i32)  [unwired: 3 out]
          n2107 = while {
            tunnel: [w3134] -> w3112
            tunnel: w3113 -> [w3131]
            stop <- w3132 continue-if-true
            n2108 = call "DMR_ImageRequestSingle.vi"("request control IN"=0, "driver handle IN"=w3131) -> ("error code OUT"=w3133:i32, "driver handle OUT"=w3134:i32)  [unwired: 2 out]
            n2109 = Equal To 0?(x=w3133) -> (x = 0?=w3132:bool)
          }
          n2110 = call "OBJ_SetI.vi"("value index IN"=0, "value IN"="Video channel", "object handle IN"=w3120) -> ()  [unwired: 2 out]
        }
        frame #3 {
          w3141 = T23 0 items=["Grayscale (U8)", "Grayscale (I16)", "Grayscale (SGL)", "Complex (CSG)", "RGB (U32)", "HSL (U32)", "RGB (U64)"] ("Image Type")
          w3149 = T23 0 items=["Grayscale (U8)", "Grayscale (I16)", "Grayscale (SGL)", "Complex (CSG)", "RGB (U32)", "HSL (U32)", "RGB (U64)"] ("Image Type")
          n2111 = call "IMAQ AVI2 Get Codec Names"() -> ("Codec Names"=w3136:string[])  [unwired: 10 in, 1 out]
          "Installed Codec Names" <- w3136
          n2112 = for "Create Greyscale map" {
            N: 256 -> [_]
            tunnel: [w3155] -> w3138 mode=indexing
            workers-P: _ -> [_]
            i -> [w3158]
            n2113 = To Unsigned Byte Integer(number=w3158) -> (unsigned 8bit integer=w3154:u8)
            n2114 = Join Numbers(hi=w3154, lo=w3154) -> ((hi.lo)=w3157:u16)
            n2115 = Join Numbers(hi=w3154, lo=w3154) -> ((hi.lo)=w3156:u16)
            n2116 = Join Numbers(hi=w3157, lo=w3156) -> ((hi.lo)=w3155:u32)
          }
          n2117 = property on="Codec choice" class="CmbBox"("Strings[]"=w3136) -> ()  [unwired: 2 in, 2 out]
          n2118 = call "IMAQ Create"("Image Name"="Scaled video", "Image Type"=w3141) -> ("New Image"=w3140:T2)  [unwired: 2 in, 2 out]
          n2119 = call "IMAQ Create"("Image Name"="Main video", "Image Type"=w3149) -> ("New Image"=w3150:T2)  [unwired: 2 in, 2 out]
          n2120 = node-c288(0 ("Processor")) -> (w3148:T27)  [unwired: 3 out]
          n2121 = Initialize Array(u32 0 ("Window Number (0...15)"), 480 ("dimension size"), 640 ("dimension size")) -> (w3143:u32[][])
          n2122 = timed-loop {
            tunnel: w3153 -> [w3175]
            tunnel: [w3174] -> w3152
            tunnel: w3150 -> [w3173]
            timing: w3148 -> [_]
            timing-out: [_] -> w3147
            tunnel: w3143 -> [w3166]
            tunnel: w3140 -> [w3164]
            tunnel: w3138 -> [w3163]
            stop <- w3165 stop-if-true
            # "This block performs the \nactual image capture."
            n2123 = node-c288() -> (→"Finished Late? [i-1]":bool)  [unwired: 5 out]
            n2124 = local read "Stop All"() -> (w3165:bool)
            n2125 = feedback #1(T40 refnum ("AVI Refnum")) -> (w3171:T40)
            n2126 = case shown="True" "New Video File" {
              tunnel: [w3188 w3189] -> w3162
              tunnel: w3171 -> [w3188 w3190]
              frame False {
              }
              frame True {
                n2127 = flat-sequence {
                  tunnel: w3190 -> [w3192]
                  tunnel: [w3194] -> w3189
                  frame #0 {
                    n2128 = local read "File open?"() -> (w3191:bool)
                    n2129 = case shown="True" w3191 {
                      tunnel: w3192 -> [_ w3193]
                      frame False {
                      }
                      frame True {
                        n2130 = call "IMAQ AVI2 Close"("AVI Refnum"=w3193) -> ()  [unwired: 10 in, 1 out]
                      }
                    }
                  }
                  frame #1 {
                    n2131 = local write "New Video File"(FALSE ("New Video File")) -> ()
                    n2132 = call "Create new save file.vi"("Ext"=".avi" ("string"), "Index In"="Video Index") -> ("Path Out"=w3197:path, "Index Out"=w3199:dbl)  [unwired: 1 in]
                    "Path Out" <- w3197
                    n2133 = local write "Video Index"(w3199) -> ()
                    n2134 = call "IMAQ AVI2 Create"("Codec"="Codec choice", "Frames Per Second"=u32 30, "AVI Path"=w3197) -> ("AVI Refnum"=w3194:T40)  [unwired: 7 in, 1 out]
                    "File open?" <- TRUE ("Files open?")
                  }
                }
              }
            }
            n2135 = feedback-in #1(w3162) -> ()
            n2136 = call "DMR_ImageRequestWaitFor.vi"("queue number IN"=0, "timeout(ms) IN"=500, "driver handle IN"=w3175) -> ("error code OUT"=w3179:i32, "request number OUT"=w3176:i32, "driver handle OUT"=w3177:i32)
            n2137 = Equal To 0?(x=w3179) -> (x = 0?=w3178:bool)
            n2138 = Reciprocal(x="Video Capture Rate (Hz)") -> (1/x=w3169:dbl)
            n2139 = Multiply(x=w3169, y=1000.0) -> (x*y=w3167:dbl)
            n2140 = case shown="True" w3178 {
              tunnel: w3177 -> [w3203 w3240]
              tunnel: w3176 -> [_ w3239]
              tunnel: [w3203 w3236] -> w3174
              tunnel: w3173 -> [_ w3222]
              tunnel: w3166 -> [_ w3225]
              tunnel: w3162 -> [_ w3205]
              tunnel: w3164 -> [_ w3219]
              tunnel: w3163 -> [_ w3218]
              frame False {
              }
              frame True {
                w3230 = u32 0 ("X-offset IN")
                n2141 = call "DMR_GetImageRequestBufferData.vi"("driver handle IN"=w3240, "request number IN"=w3239) -> ("width OUT"=w3229:i32, "height OUT"=w3228:i32, "driver handle OUT"=w3235:i32, "request number OUT"=w3234:i32, "bytes per pixel OUT"=w3231:i32)  [unwired: 13 out]
                n2142 = call "DMR_GetImageRequestBufferImageData.vi"("driver handle IN"=w3235, "request number IN"=w3234, "bytes per pixel IN"=w3231, "X-offset IN"=w3230, "Y-offset IN"=w3230, "height IN"=w3228, "width IN"=w3229) -> ("driver handle OUT"=w3233:u32, "request number OUT"=w3232:u32, "image OUT"=w3211:u32[][])  [unwired: 10 out]